vi "InsertDeadTimeSpectrogram.vi"() -> ()   [LabVIEW 2022 SP3]
panel:
  out "Spectorgram at marker 3":sgl[][](graph)
  out "Spectorgram at marker 2":dbl[][](graph)
  out "size(s) 2":i32[](array[numeric])
  out "size(s)":i32[](array[numeric])
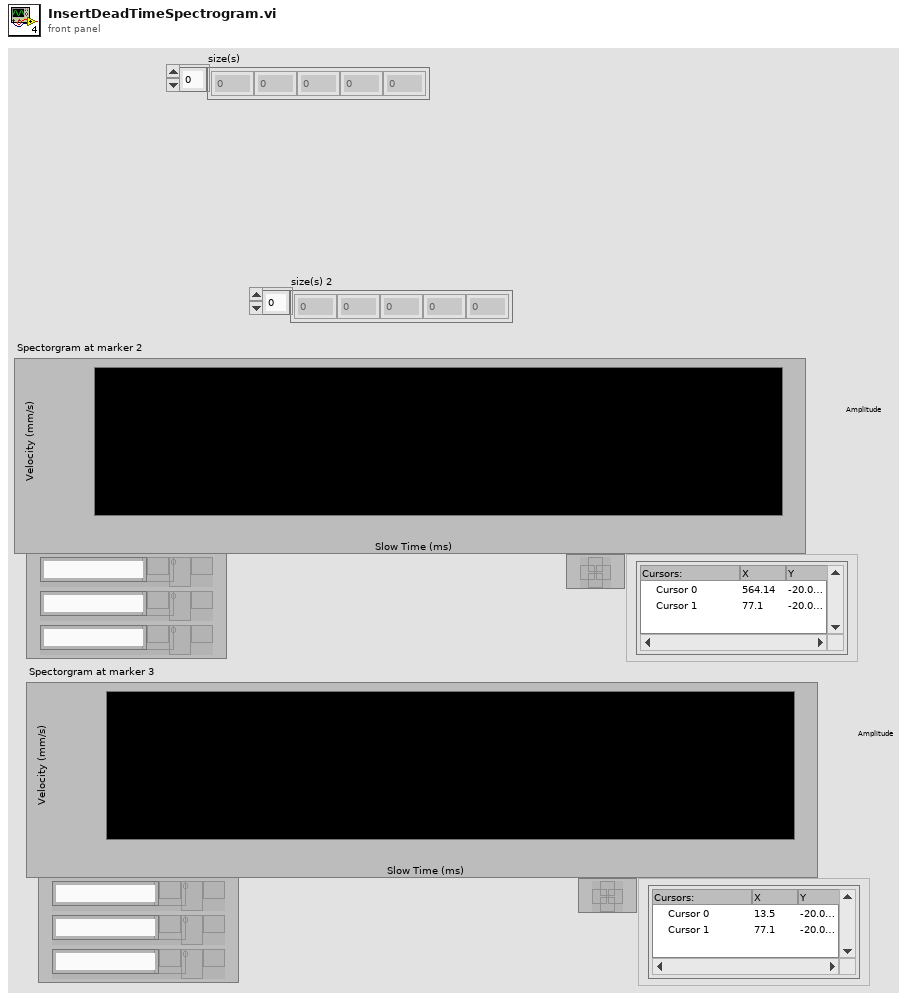
[diagram p1: front panel]
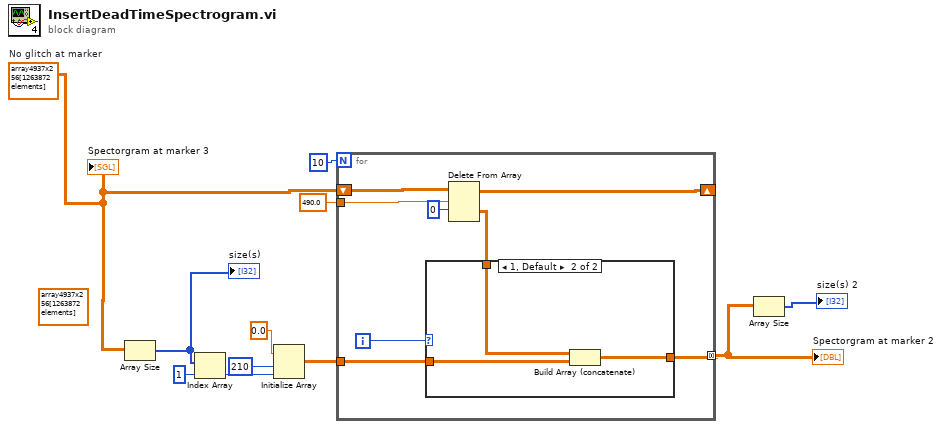
[diagram p0: block diagram]
diagram:
  w1 = sgl[][] array4937x256[1263872 elements]  # No glitch at marker
  (unwired) sgl[][] array4937x256[1263872 elements] ("Spectorgram at marker")
  n1 = Array Size(array=w1) -> (size(s)=w10:i32[])
  "size(s)" <- w10
  n2 = Index Array(array=w10, index=1) -> (element=w8:i32)
  n3 = Initialize Array(0.0 ("element"), 210 ("dimension size"), w8) -> (w5:dbl[][])
  n4 = for {
    N: 10 -> [_]
    shift-right: [w13] -> _
    shift-left: w1 -> [w18]
    tunnel: 490.0 ("element") -> [w17]
    tunnel: [w16] -> w4 mode=concatenating
    tunnel: w5 -> [w15]
    i -> [w19]
    n5 = Delete From Array(array=w18, length=w17, index (row)=0) -> (deleted portion=w14:sgl[][], array with subset deleted=w13:sgl[][])  [unwired: 1 in]
    n6 = case shown="1, Default" w19 {
      tunnel: [w20 w21] -> w16
      tunnel: w14 -> [w20 w23]
      tunnel: w15 -> [_ w22]
      frame 0 {
      }
      frame 1, Default {
        n7 = Build Array (concatenate)(w23, w22) -> (w21:dbl[][])
      }
    }
  }
  "Spectorgram at marker 2" <- w4
  n8 = Array Size(array=w4) -> (size(s)=→"size(s) 2":i32[])
  "Spectorgram at marker 3" <- w1
